vi "HFRR ADV v041.vi"() -> ()   [LabVIEW 2025] (continued)
                  frame False {
                  }
                  frame True {
                    w3298 = ";" ("Substring")
                    # "Pid out/\nFreq response value"
                    n2711 = local write "act save time"(w3344) -> ()
                    n2712 = local read "FILE"() -> (w3292:string)
                    n2713 = call "file check.vi"("file name in"=w3292) -> ("error out"=w3295:errorcluster, "file name out"=w3290:string)  [unwired: 9 in]
                    n2714 = local read "LVDT STROKE"() -> (w3287:dbl)
                    n2715 = local read "Add up Stroke"() -> (w3285:dbl)
                    n2716 = call "FILE PATH CREATION.vi"("error in"=w3295, "FILE NAME :"=w3290) -> ("FILE OUT"=w3293:path)  [unwired: 8 in, 1 out]
                    n2717 = local read "STROKE Initialize"() -> (w3280:bool)
                    n2718 = Concatenate Strings(w3290, ".dgf" ("Substring")) -> (w3294:string)
                    n2719 = Subtract(x=w3287, y=w3285) -> (x-y=w3286:dbl)
                    n2720 = Absolute Value(x=w3286) -> (abs(x)=w3283:dbl)
                    n2721 = local read "FF 2"() -> (→"Frictional Force ( N )" →"Frictional Force ( N )":dbl)
                    n2722 = Build Path(base path=w3293, name or relative path=w3294) -> (appended path=w3289:path)
                    n2723 = flat-sequence {
                      tunnel: w3283 -> [w3349]
                      tunnel: [w3348] -> w3281
                      tunnel: w3280 -> [w3346]
                      tunnel: [w3351] -> w3282
                      tunnel: w3281 -> [w3351]
                      frame #0 {
                        n2724 = call <vilib>:"Mean PtByPt.vi"("x"=w3349, "sample length"="STROKE FILTER", "initialize"=w3346) -> ("mean"=w3348:dbl)  [unwired: 1 in, 1 out]
                      }
                      frame #1 {
                        "STROKE Initialize" <- FALSE ("STROKE Initialize")
                      }
                    }
                    n2725 = local read "COF 2"() -> (w3303:dbl)
                    "Coefficient of Friction" <- w3303
                    "COF 4" <- w3303
                    "Coefficient of Friction" <- w3303
                    n2726 = local read "TEMP"() -> (w3306:dbl)
                    "Temperature ( Deg C )" <- w3306
                    n2727 = local read "Humidity ( %RH )"() -> (w3305:dbl)
                    n2728 = local read "Frequency ( Hz )"() -> (w3312:dbl)
                    n2729 = local read "LVDT STROKE DISPLAY"() -> (w3284:dbl)
                    n2730 = local read "Elapsed time"() -> (w3337:dbl)
                    n2731 = local read "AIR TEMP"() -> (w3310:dbl)
                    n2732 = local read "PID-out"() -> (w3315:dbl)
                    n2733 = local write "Temperature ( Deg C )"(w3306) -> ()
                    n2734 = Number To Fractional String(number=w3284, width (-)=i16 9 ("precision (6)"), precision (6)=i16 6) -> (F-format string=w3330:string)  [unwired: 1 in]
                    n2735 = Number To Fractional String(number=w3310, width (-)=i16 9 ("precision (6)"), precision (6)=i16 3) -> (F-format string=w3329:string)  [unwired: 1 in]
                    n2736 = Number To Fractional String(number=w3306, width (-)=i16 9 ("precision (6)"), precision (6)=i16 3) -> (F-format string=w3326:string)  [unwired: 1 in]
                    n2737 = Number To Fractional String(number=w3305, width (-)=i16 9 ("precision (6)"), precision (6)=i16 3) -> (F-format string=w3323:string)  [unwired: 1 in]
                    n2738 = Number To Fractional String(number=0.0, width (-)=i16 9 ("precision (6)"), precision (6)=i16 3) -> (F-format string=w3320:string)  [unwired: 1 in]
                    n2739 = Number To Fractional String(number=w3315, width (-)=i16 9 ("precision (6)"), precision (6)=i16 3) -> (F-format string=w3316:string)  [unwired: 1 in]
                    n2740 = Number To Fractional String(number=w3312, width (-)=i16 9 ("precision (6)"), precision (6)=i16 3) -> (F-format string=w3311:string)  [unwired: 1 in]
                    n2741 = Number To Fractional String(number=w3303, width (-)=i16 9 ("precision (6)"), precision (6)=i16 6) -> (F-format string=w3338:string)  [unwired: 1 in]
                    n2742 = Number To Fractional String(number=w3337, width (-)=i16 14 ("precision (6)"), precision (6)=i16 3) -> (F-format string=w3339:string)  [unwired: 1 in]
                    n2743 = Bundle("y"=1.02, "LVDT STROKE DISPLAY"=w3284, "y"=0.98) -> (w3304:T31)  [unwired: 1 in]
                    n2744 = Number To Fractional String(number="Ambient Humidity :", width (-)=i16 9 ("precision (6)"), precision (6)=i16 6) -> (F-format string=w3296:string)  [unwired: 1 in]
                    n2745 = local read "RUN"() -> (w3302:bool)
                    n2746 = case shown="True" w3302 {
                      tunnel: w3304 -> [_ w3355]
                      tunnel: w3284 -> [_ w3354]
                      tunnel: w3284 -> [_ w3352]
                      tunnel: w3284 -> [_ w3353]
                      frame False {
                      }
                      frame True {
                        "Stroke ( mm )" <- w3355
                        "Stroke ( mm )" <- w3355
                        "Stroke 4" <- w3354
                        "Stroke 3" <- w3352
                        "Stroke 2" <- w3353
                        "measured_stroke" <- w3352
                      }
                    }
                    n2747 = Concatenate Strings(w3339, w3298, w3338, w3298, w3330, w3298, w3329, w3298, w3326, w3298, w3323, w3298, w3320, w3298, w3316, w3298, w3311, w3298, w3296, "\r") -> (w3336:string)
                    n2748 = call <vilib>:"Write Characters To File.vi"("append to file? (new file:F)"=TRUE, "character string"=w3336, "file path (dialog if empty)"=w3289) -> ()  [unwired: 2 in, 1 out]
                    "refresh flag" <- TRUE ("refresh flag")
                    "LVDT STROKE Actual" <- w3282
                  }
                }
                n2749 = case shown="True" w3204 {
                  tunnel: w3214 -> [_ w3240]
                  tunnel: w3219 -> [_ w3250]
                  tunnel: [0.0 w3246] -> _
                  tunnel: w3213 -> [_ w3245]
                  tunnel: [0.0 w3244] -> _
                  tunnel: w3203 -> [_ w3244]
                  tunnel: w3217 -> [w3233 _]
                  frame False {
                    n2750 = local write "acq timer"(w3233) -> ()
                    n2751 = local write "Test Duration Status"(0.0 ("Test Duration Status")) -> ()
                  }
                  frame True {
                    n2752 = local read "Set Hz"() -> (w3247:dbl)
                    n2753 = local write "Elapsed time"(w3240) -> ()
                    n2754 = local read "test time"() -> (w3239:dbl)
                    n2755 = Multiply(x=w3250, y=w3247) -> (x*y=w3249:dbl)
                    n2756 = case shown="False" w3245 {
                      tunnel: w3249 -> [w3251 _]
                      tunnel: [w3251 1.0] -> w3246
                      frame False {
                        n2757 = local write "Cycles elapsed"(w3251) -> ()
                      }
                      frame True {
                      }
                    }
                    n2758 = Greater?(x=w3240, y=w3239) -> (0:w3248:bool)
                    n2759 = Subtract(x=w3239, y=w3240) -> (x-y=w3238:dbl)
                    n2760 = Multiply(x=w3238, y=60.0) -> (x*y=w3237:dbl)
                    n2761 = local write "Time Remaining"(w3237) -> ()
                    n2762 = local write "Remaining Time"(w3237) -> ()
                    n2763 = case shown="True" w3248 {
                      frame False {
                      }
                      frame True {
                        n2764 = stacked-sequence {
                          frame #0 {
                            w3256 = T19."Enabled" ("Disabled")
                            w3255 = FALSE ("TEST FILE NAM,E SAVED")
                            w3257 = "" ("FILE")
                            w3258 = TRUE ("Visible")
                            n2765 = local write "Humidity"(FALSE ("Humidity")) -> ()
                            n2766 = local write "RUN"(FALSE ("OK Button 2")) -> ()
                            n2767 = local write "Heater Button"(FALSE ("Heater Button")) -> ()
                            n2768 = local write "Auto Start Test"(FALSE ("Auto Start Test")) -> ()
                            n2769 = local write "TestCompFlg"(TRUE ("StpFlg")) -> ()
                            n2770 = local read "Humidity ( %RH )"() -> (→"Rh After":dbl)
                            n2771 = property on="STOP 2" class="Bool (strict)"("Disabled"=u8 0) -> ()  [unwired: 2 in, 2 out]
                            n2772 = local read "EVENT LOG"() -> (w3263:string)
                            n2773 = call "Event Log.vi"("Content"="Test Completed", "EVENT LOG"=w3263) -> ("EVENT LOG"=w3262:string)  [unwired: 8 in, 1 out]
                            n2774 = property on="RUN" class="Bool (strict)"("Visible"=w3258) -> ()  [unwired: 2 in, 2 out]
                            n2775 = property on="Auto Start Test" class="Bool (strict)"("Visible"=w3258) -> ()  [unwired: 2 in, 2 out]
                            n2776 = local write "Batch Ref Num :"(w3257) -> ()
                            n2777 = local write "FILE"(w3257) -> ()
                            n2778 = local write "EVENT LOG"(w3262) -> ()
                            n2779 = local write "TEST FILE NAM,E SAVED"(w3255) -> ()
                            n2780 = local write "Fuel Discription :"(w3257) -> ()
                            n2781 = local write "START TEMP"(w3255) -> ()
                            n2782 = local write "Remarks :"(w3257) -> ()
                            n2783 = local write "Main Dashboard Buttons"(T1."Imaging" ("Main Dashboard Buttons")) -> ()
                            n2784 = local write "Main Tab"(T2."Adv Scar" ("Main Tab")) -> ()
                            n2785 = property on="FRICVALZ 2" class="Bool (strict)"("DisabledEnum"=w3256) -> ()  [unwired: 2 in, 2 out]
                            n2786 = property on="FRICVALZ 3" class="Bool (strict)"("DisabledEnum"=w3256) -> ()  [unwired: 2 in, 2 out]
                            n2787 = property on="FRICVALZ 4" class="Bool (strict)"("DisabledEnum"=w3256) -> ()  [unwired: 2 in, 2 out]
                          }
                          frame #1 {
                            n2788 = Wait (ms)(milliseconds to wait=u32 1500) -> ()  [unwired: 1 out]
                          }
                          frame #2 {
                            n2789 = local write "Due Write"("VC;0") -> ()
                          }
                          frame #3 {
                            n2790 = Wait (ms)(milliseconds to wait=u32 1500) -> ()  [unwired: 1 out]
                          }
                          frame #4 {
                            n2791 = local write "Due Write"("VC;0") -> ()
                          }
                          frame #5 {
                            n2792 = Wait (ms)(milliseconds to wait=u32 1500) -> ()  [unwired: 1 out]
                          }
                          frame #6 {
                            n2793 = local write "Due Write"("ST;0") -> ()
                          }
                          frame #7 {
                            n2794 = local write "measured_stroke"(0.0 ("measured_stroke")) -> ()
                            n2795 = Wait (ms)(milliseconds to wait=u32 1500) -> ()  [unwired: 1 out]
                          }
                          frame #8 {
                            n2796 = local write "Due Write"("HE;0") -> ()
                            n2797 = local write "Humidity 2"(TRUE ("Humidity")) -> ()
                          }
                        }
                      }
                    }
                    n2798 = Divide(x=w3240, y=w3239) -> (x/y=w3243:dbl)
                    n2799 = Multiply(x=w3243, y=100.0) -> (x*y=w3241:dbl)
                    n2800 = local write "Test Duration Status"(w3241) -> ()
                  }
                }
              }
              frame #2 {
                n2801 = case shown="True" "Heater Button" {
                  tunnel: [0.0 ("output") w3378] -> w3356
                  frame False {
                    w3359 = TRUE ("tmpchk")
                    n2802 = local read "TEMP"() -> (w3360:dbl)
                    n2803 = local write "Temp ini"(w3360) -> ()
                    n2804 = local write "Reset 4"(w3359) -> ()
                    n2805 = local write "tmpchk"(w3359) -> ()
                    n2806 = local write "reinit"(TRUE ("reinit")) -> ()
                    n2807 = local write "manual temp log"(TRUE ("manual temp log")) -> ()
                  }
                  frame True {
                    # "Logic to turn off\nthe heater when \ntemp is not rising.\nTime - 60 sec\nDelta t- 5°c"
                    n2808 = local read "Temp ini"() -> (w3367:dbl)
                    n2809 = local read "Auto Start Test"() -> (w3363:bool)
                    n2810 = Less?(x=w3367, y=53.0) -> (x < y?=w3365:bool)
                    n2811 = case shown="False" w3363 {
                      frame False {
                        n2812 = local read "Set Temp"() -> (w3387:dbl)
                        n2813 = local read "TEMP"() -> (w3386:dbl)
                        n2814 = Subtract(x=w3387, y=w3386) -> (x-y=w3385:dbl)
                        n2815 = Absolute Value(x=w3385) -> (abs(x)=w3384:dbl)
                        n2816 = Less?(x=w3384, y=0.5) -> (x < y?=w3382:bool)
                        n2817 = case shown="True" w3382 {
                          tunnel: "manual temp log" -> [_ w3388]
                          frame False {
                          }
                          frame True {
                            n2818 = case shown="True" w3388 {
                              selector: w3388 -> [_ w3389]
                              frame False {
                              }
                              frame True {
                                # "#Event log"
                                n2819 = Not(x=w3389) -> (.not. x?=w3390:bool)
                                n2820 = local write "manual temp log"(w3390) -> ()
                                n2821 = local read "EVENT LOG"() -> (w3393:string)
                                n2822 = call "Event Log.vi"("Content"="Target Temperature reached", "EVENT LOG"=w3393) -> ("EVENT LOG"=w3392:string)  [unwired: 8 in, 1 out]
                                n2823 = local write "EVENT LOG"(w3392) -> ()
                              }
                            }
                          }
                        }
                      }
                      frame True {
                        n2824 = local write "manual temp log"(TRUE ("manual temp log")) -> ()
                      }
                    }
                    n2825 = And(x="tmpchk", y=w3365) -> (x .and. y?=w3368:bool)
                    n2826 = case shown="True" w3368 {
                      frame False {
                      }
                      frame True {
                        n2827 = call "Elapsed Time8"("Time Target (s)"=300.0, "Reset"="Reset 4") -> ("Time has Elapsed"=w3395:bool)  [unwired: 10 in, 7 out]
                        n2828 = flat-sequence {
                          tunnel: w3395 -> [_]
                          frame #0 {
                            n2829 = local write "Reset 4"(FALSE ("Reset 4")) -> ()
                          }
                        }
                        n2830 = case shown="True" w3395 {
                          frame False {
                          }
                          frame True {
                            n2831 = local read "Temp ini"() -> (w3402:dbl)
                            n2832 = Add(x=w3402, y=5.0) -> (x+y=w3400:dbl)
                            n2833 = local read "TEMP"() -> (w3403:dbl)
                            n2834 = Greater?(x=w3403, y=w3400) -> (0:w3401:bool)
                            n2835 = case shown="False" w3401 {
                              frame False {
                                n2836 = local write "Heater Button"(FALSE ("Heater Button")) -> ()
                              }
                              frame True {
                                n2837 = local write "tmpchk"(FALSE ("tmpchk")) -> ()
                              }
                            }
                          }
                        }
                      }
                    }
                    n2838 = local read "Set Temp"() -> (w3376:dbl)
                    n2839 = local read "TEMP"() -> (w3370:dbl)
                    n2840 = call-poly <vilib>:"PID.vi"("reinitialize? (F)"="reinit", "dt (s)"=-1.0, "process variable"=w3370, "setpoint"=w3376) -> ("output"=w3373:dbl)  [unwired: 6 in, 1 out]
                    n2841 = Subtract(x=w3376, y=w3370) -> (x-y=w3377:dbl)
                    n2842 = Add(x=w3376, y=0.5) -> (x+y=w3374:dbl)
                    n2843 = Greater Or Equal?(x=w3370, y=w3374) -> ()  [unwired: 1 out]
                    n2844 = Select(t=0.0, s=FALSE, f=w3373) -> (s? t:f=w3372:dbl)
                    "PID output" <- w3372
                    n2845 = flat-sequence {
                      tunnel: w3372 -> [w3406]
                      tunnel: [w3406] -> w3378
                      frame #0 {
                        n2846 = local write "reinit"(FALSE ("reinit")) -> ()
                      }
                    }
                    n2847 = Bundle(w3377, "output"=w3372, "TEMP"=w3370) -> ()  [unwired: 1 in, 1 out]
                  }
                }
                "PID-out" <- w3356
              }
              frame #3 {
                n2848 = local read "TEMP"() -> (w3408:dbl)
                n2849 = Greater Or Equal?(x=w3408, y="Set Temp 2") -> (x >= y?=w3413:bool)
                n2850 = case shown="True" w3413 {
                  tunnel: [FALSE TRUE] -> w3411
                  frame False {
                  }
                  frame True {
                  }
                }
                "Status 13" <- w3411
                n2851 = And(x=w3411, y="trip1 8") -> (x .and. y?=w3410:bool)
                n2852 = case shown="True" w3410 {
                  frame False {
                    n2853 = local write "Heater Trip Temp"(TRUE ("Heater Trip Temp")) -> ()
                  }
                  frame True {
                    w3416 = FALSE ("OK Button 2")
                    n2854 = case shown="True" "Heater Trip Temp" {
                      selector: "Heater Trip Temp" -> [_ w3418]
                      frame False {
                      }
                      frame True {
                        n2855 = Not(x=w3418) -> (.not. x?=w3417:bool)
                        n2856 = local read "EVENT LOG"() -> (w3421:string)
                        n2857 = local write "Heater Trip Temp"(w3417) -> ()
                        n2858 = call "Event Log.vi"("Content"="Heater Trip", "EVENT LOG"=w3421) -> ("EVENT LOG"=w3420:string)  [unwired: 8 in, 1 out]
                        n2859 = local write "EVENT LOG"(w3420) -> ()
                      }
                    }
                    n2860 = local write "RUN"(w3416) -> ()
                    n2861 = property on="Auto Start Test" class="Bool (strict)"("Value"=w3416) -> ()  [unwired: 2 in, 2 out]
                    n2862 = local write "Heater Button"(w3416) -> ()
                  }
                }
              }
            }
            n2863 = case shown="False" w3127 {
              frame False {
                n2864 = disable-structure shown="Disabled" {
                  frame Disabled {
                    n2865 = stacked-sequence {
                      frame #0 {
                        n2866 = local write "RUN"(FALSE ("OK Button 2")) -> ()
                      }
                      frame #1 {
                      }
                    }
                  }
                  frame Enabled {
                  }
                }
              }
              frame True {
              }
            }
          }
        }
        n2867 = local read "Reset Graph"() -> (w3024:bool)
        n2868 = case shown="True" w3024 {
          selector: w3024 -> [_ w3041]
          frame False {
          }
          frame True {
            w3055 = 0.0 ("X Scale.Range:Maximum")
            n2869 = Not(x=w3041) -> (.not. x?=w3040:bool)
            n2870 = local write "Reset Graph"(w3040) -> ()
            n2871 = property on="Electrical Contact Resistance ( % )" class="WFChart (strict)"("XScale.Maximum"=600.0 ("X Scale.Range:Maximum"), "XScale.Minimum"=0.0 ("X Scale.Range:Minimum"), "YScale.Maximum"=100.0 ("Y Scale.Range:Maximum"), "YScale.Minimum"=0.0 ("Y Scale.Range:Minimum")) -> ()  [unwired: 2 in, 2 out]
            n2872 = property on="Frictional Force ( N )" class="WFChart (strict)"("XScale.Maximum"=600.0 ("X Scale.Range:Maximum"), "XScale.Minimum"=0.0 ("X Scale.Range:Minimum"), "YScale.Maximum"=100.0 ("Y Scale.Range:Maximum"), "YScale.Minimum"=0.0 ("Y Scale.Range:Minimum")) -> ()  [unwired: 2 in, 2 out]
            n2873 = property on="Temperature ( Deg C )" class="WFChart (strict)"("XScale.Maximum"=600.0 ("X Scale.Range:Maximum"), "XScale.Minimum"=0.0 ("X Scale.Range:Minimum"), "YScale.Maximum"=100.0 ("Y Scale.Range:Maximum"), "YScale.Minimum"=0.0 ("Y Scale.Range:Minimum")) -> ()  [unwired: 2 in, 2 out]
            n2874 = property on="Stroke ( mm )" class="WFChart (strict)"("XScale.Maximum"=600.0 ("X Scale.Range:Maximum"), "XScale.Minimum"=0.0 ("X Scale.Range:Minimum"), "YScale.Maximum"=100.0 ("Y Scale.Range:Maximum"), "YScale.Minimum"=0.0 ("Y Scale.Range:Minimum")) -> ()  [unwired: 2 in, 2 out]
            n2875 = property on="Coefficient of Friction" class="WFChart (strict)"("XScale.Maximum"=600.0 ("X Scale.Range:Maximum"), "XScale.Minimum"=0.0 ("X Scale.Range:Minimum"), "YScale.Maximum"=100.0 ("Y Scale.Range:Maximum"), "YScale.Minimum"=0.0 ("Y Scale.Range:Minimum")) -> ()  [unwired: 2 in, 2 out]
            n2876 = property on="Electrical Contact Resistance ( % )" class="WFChart (strict)"("XScale.Minimum"=0.0 ("X Scale.Range:Minimum"), "XScale.Maximum"=600.0 ("X Scale.Range:Maximum"), "YScale.Minimum"=0.0 ("Y Scale.Range:Minimum"), "YScale.Maximum"=100.0 ("Y Scale.Range:Maximum")) -> ()  [unwired: 2 in, 2 out]
            n2877 = property on="Temperature ( Deg C )" class="WFChart (strict)"("XScale.Minimum"=0.0 ("X Scale.Range:Minimum"), "XScale.Maximum"=600.0 ("X Scale.Range:Maximum"), "YScale.Minimum"=0.0 ("Y Scale.Range:Minimum"), "YScale.Maximum"=100.0 ("Y Scale.Range:Maximum")) -> ()  [unwired: 2 in, 2 out]
            n2878 = property on="Coefficient of Friction" class="WFChart (strict)"("XScale.Minimum"=0.0 ("X Scale.Range:Minimum"), "XScale.Maximum"=600.0 ("X Scale.Range:Maximum"), "YScale.Maximum"=1.0 ("X Scale.Range:Minimum"), "YScale.Minimum"=0.0 ("X Scale.Range:Minimum")) -> ()  [unwired: 2 in, 2 out]
            n2879 = property on="Frictional Force ( N )" class="WFChart (strict)"("XScale.Maximum"=600.0 ("X Scale.Range:Maximum"), "XScale.Minimum"=w3055, "YScale.Maximum"=10.0 ("Y Scale.Range:Maximum"), "YScale.Minimum"=w3055) -> ()  [unwired: 2 in, 2 out]
            n2880 = property on="Stroke ( mm )" class="WFChart (strict)"("XScale.Maximum"=600.0 ("X Scale.Range:Maximum"), "XScale.Minimum"=0.0 ("X Scale.Range:Minimum"), "YScale.Maximum"=100.0 ("Y Scale.Range:Maximum"), "YScale.Minimum"=0.0 ("Y Scale.Range:Minimum")) -> ()  [unwired: 2 in, 2 out]
          }
        }
      }
      frame "Compare Files" {
        # "Elapsed time\ncof\nstroke\nAir temp\nTemp\nHumidity"
        n2881 = case shown="True" "RSTV1 2" {
          frame False {
          }
          frame True {
            n2882 = property on="Humidity ( %RH )" class="XYGraph (strict)"("Y Scale.Display Format:Precision"=u8 0 ("Y Scale.Format & Precision:Precision")) -> ()  [unwired: 2 in, 2 out]
            n2883 = property on="Humidity ( %RH )" class="XYGraph (strict)"("X Scale.Range:Minimum"=0.0, "X Scale.Range:Maximum"=75.0, "Y Scale.Range:Minimum"=48.0, "Y Scale.Range:Maximum"=58.0) -> ()  [unwired: 2 in, 2 out]
          }
        }
        n2884 = case shown="True" "RST CP 2" {
          frame False {
          }
          frame True {
            n2885 = property on="XY Graph 13" class="XYGraph (strict)"("Y Scale.Display Format:Precision"=u8 0 ("Y Scale.Format & Precision:Precision")) -> ()  [unwired: 2 in, 2 out]
            n2886 = property on="XY Graph 13" class="XYGraph (strict)"("X Scale.Range:Minimum"=0.0, "X Scale.Range:Maximum"=75.0, "Y Scale.Range:Minimum"=0.0, "Y Scale.Range:Maximum"=100.0) -> ()  [unwired: 2 in, 2 out]
          }
        }
        n2887 = case shown="True" "RST CP" {
          frame False {
          }
          frame True {
            n2888 = property on="Sample Temperature ( °C )" class="XYGraph (strict)"("Y Scale.Display Format:Precision"=u8 2 ("Y Scale.Format & Precision:Precision")) -> ()  [unwired: 2 in, 2 out]
            n2889 = property on="Sample Temperature ( °C )" class="XYGraph (strict)"("X Scale.Range:Minimum"=0.0, "X Scale.Range:Maximum"=75.0, "Y Scale.Range:Minimum"=58.0, "Y Scale.Range:Maximum"=62.0) -> ()  [unwired: 2 in, 2 out]
          }
        }
        n2890 = case shown="True" "RSTV1 3" {
          frame False {
          }
          frame True {
            n2891 = property on="Air Temperature  ( °C )" class="XYGraph (strict)"("Y Scale.Display Format:Precision"=u8 2 ("Y Scale.Format & Precision:Precision")) -> ()  [unwired: 2 in, 2 out]
            n2892 = property on="Air Temperature  ( °C )" class="XYGraph (strict)"("X Scale.Range:Minimum"=0.0 ("Y Scale.Range:Minimum"), "X Scale.Range:Maximum"=75.0 ("Y Scale.Range:Maximum"), "Y Scale.Range:Minimum"=20.0 ("X Scale.Range:Minimum"), "Y Scale.Range:Maximum"=26.0 ("X Scale.Range:Maximum")) -> ()  [unwired: 2 in, 2 out]
          }
        }
        n2893 = case shown="True" "RSTV1 4" {
          frame False {
          }
          frame True {
            n2894 = property on="Stroke ( mm )" class="XYGraph (strict)"("Y Scale.Display Format:Precision"=u8 2 ("Y Scale.Format & Precision:Precision")) -> ()  [unwired: 2 in, 2 out]
            n2895 = property on="Stroke ( mm )" class="XYGraph (strict)"("X Scale.Range:Minimum"=0.0 ("Y Scale.Range:Maximum"), "X Scale.Range:Maximum"=75.0 ("X Scale.Range:Minimum"), "Y Scale.Range:Minimum"=0.98, "Y Scale.Range:Maximum"=1.02) -> ()  [unwired: 2 in, 2 out]
          }
        }
        n2896 = case shown="True" "rstv2" {
          frame False {
          }
          frame True {
            n2897 = property on="Coefficient Of Friction" class="XYGraph (strict)"("Y Scale.Display Format:Precision"=u8 3 ("Y Scale.Format & Precision:Precision")) -> ()  [unwired: 2 in, 2 out]
            n2898 = property on="Coefficient Of Friction" class="XYGraph (strict)"("X Scale.Range:Minimum"=0.0 ("Y Scale.Range:Maximum"), "X Scale.Range:Maximum"=75.0, "Y Scale.Range:Minimum"=0.0, "Y Scale.Range:Maximum"=1.0 ("X Scale.Range:Minimum")) -> ()  [unwired: 2 in, 2 out]
          }
        }
        n2899 = case shown="True" "RST CP 3" {
          frame False {
          }
          frame True {
            n2900 = property on="Air Temp ( °C ) vs Humidity ( % RH )" class="XYGraph (strict)"("X Scale.Range:Minimum"=18.0, "X Scale.Range:Maximum"=28.0 ("X Scale.Range:Minimum"), "Y Scale.Range:Minimum"=30.0 ("X Scale.Range:Minimum"), "Y Scale.Range:Maximum"=70.0 ("X Scale.Range:Minimum")) -> ()  [unwired: 2 in, 2 out]
          }
        }
        n2901 = case shown="True" "OPEN 1" {
          frame False {
          }
          frame True {
            (unwired) 0  # existing file
            w3697 = "Choose a datalog file to open"  # prompt
            n2902 = local write "OPEN 1"(FALSE ("OPEN 1")) -> ()
            n2903 = String To Path(string="C:\\LAB-IQ\\Data\\") -> (path=w3682:path)
            n2904 = File Dialog(6:"*.dgf" ("pattern"), 7:w3697, 11:w3682) -> (0:w3680:errorcluster, 3:w3688:path)  [unwired: 4 in, 2 out]
            n2905 = Unbundle(w3680) -> ()  [unwired: 3 out]
            n2906 = Strip Path(path=w3688) -> (name=w3687:string)  [unwired: 1 out]
            n2907 = Path To String(path=w3688) -> (string=w3683:string)
            "string1" <- w3683
            n2908 = Match Pattern(string=w3687, regular expression=".dgf") -> (before substring=→"String Control":string)  [unwired: 1 in, 3 out]
            n2909 = Match Pattern(string=w3683, regular expression=".dgf" ("substring (\"\")")) -> (before substring=w3693:string)  [unwired: 1 in, 3 out]
            n2910 = Concatenate Strings(w3693, ".duf" ("Substring")) -> (w3689:string)
            n2911 = String To Path(string=w3689) -> (path=w3694:path)
            n2912 = call <vilib>:"Read Characters From File.vi"("file path (dialog if empty)"=w3694, "start of read offset (chars.:0)"=60 ("start of read offset (chars.: 0)")) -> ("character string"=→"String Control 2":string)  [unwired: 4 in, 3 out]
          }
        }
        n2913 = case shown="True" "OPEN 2" {
          frame False {
          }
          frame True {
            (unwired) 0  # existing file
            w3715 = "Choose a datalog file to open"  # prompt
            n2914 = local write "OPEN 2"(FALSE ("OPEN 1")) -> ()
            n2915 = String To Path(string="C:\\LAB-IQ\\Data\\") -> (path=w3700:path)
            n2916 = File Dialog(6:"*.dgf" ("pattern"), 7:w3715, 11:w3700) -> (0:w3698:errorcluster, 3:w3706:path)  [unwired: 4 in, 2 out]
            n2917 = Unbundle(w3698) -> ()  [unwired: 3 out]
            n2918 = Strip Path(path=w3706) -> (name=w3704:string)  [unwired: 1 out]
            n2919 = Path To String(path=w3706) -> (string=w3701:string)
            "string1 2" <- w3701
            n2920 = Match Pattern(string=w3704, regular expression=".dgf") -> (before substring=→"String Control 3":string)  [unwired: 1 in, 3 out]
            n2921 = Match Pattern(string=w3701, regular expression=".dgf" ("substring (\"\")")) -> (before substring=w3712:string)  [unwired: 1 in, 3 out]
            n2922 = Concatenate Strings(w3712, ".duf" ("Substring")) -> (w3709:string)
            n2923 = String To Path(string=w3709) -> (path=w3707:path)
            n2924 = call <vilib>:"Read Characters From File.vi"("file path (dialog if empty)"=w3707, "start of read offset (chars.:0)"=60 ("start of read offset (chars.: 0)")) -> ("character string"=→"String Control 4":string)  [unwired: 4 in, 3 out]
          }
        }
        n2925 = case shown="True" "OPEN 3" {
          frame False {
          }
          frame True {
            (unwired) 0  # existing file
            w3733 = "Choose a datalog file to open"  # prompt
            n2926 = local write "OPEN 3"(FALSE ("OPEN 1")) -> ()
            n2927 = String To Path(string="C:\\LAB-IQ\\Data\\") -> (path=w3718:path)
            n2928 = File Dialog(6:"*.dgf" ("pattern"), 7:w3733, 11:w3718) -> (0:w3716:errorcluster, 3:w3724:path)  [unwired: 4 in, 2 out]
            n2929 = Unbundle(w3716) -> ()  [unwired: 3 out]
            n2930 = Strip Path(path=w3724) -> (name=w3722:string)  [unwired: 1 out]
            n2931 = Path To String(path=w3724) -> (string=w3719:string)
            "string1 3" <- w3719
            n2932 = Match Pattern(string=w3722, regular expression=".dgf") -> (before substring=→"String Control 5":string)  [unwired: 1 in, 3 out]
            n2933 = Match Pattern(string=w3719, regular expression=".dgf" ("substring (\"\")")) -> (before substring=w3729:string)  [unwired: 1 in, 3 out]
            n2934 = Concatenate Strings(w3729, ".duf" ("Substring")) -> (w3726:string)
            n2935 = String To Path(string=w3726) -> (path=w3730:path)
            n2936 = call <vilib>:"Read Characters From File.vi"("file path (dialog if empty)"=w3730, "start of read offset (chars.:0)"=60 ("start of read offset (chars.: 0)")) -> ("character string"=→"String Control 6":string)  [unwired: 4 in, 3 out]
          }
        }
        n2937 = case shown="True" "OPEN 4" {
          frame False {
          }
          frame True {
            (unwired) 0  # existing file
            w3751 = "Choose a datalog file to open"  # prompt
            n2938 = local write "OPEN 4"(FALSE ("OPEN 1")) -> ()
            n2939 = String To Path(string="C:\\LAB-IQ\\Data\\") -> (path=w3736:path)
            n2940 = File Dialog(6:"*.dgf" ("pattern"), 7:w3751, 11:w3736) -> (0:w3734:errorcluster, 3:w3742:path)  [unwired: 4 in, 2 out]
            n2941 = Unbundle(w3734) -> ()  [unwired: 3 out]
            n2942 = Strip Path(path=w3742) -> (name=w3740:string)  [unwired: 1 out]
            n2943 = Path To String(path=w3742) -> (string=w3737:string)
            "string1 4" <- w3737
            n2944 = Match Pattern(string=w3740, regular expression=".dgf") -> (before substring=→"String Control 7":string)  [unwired: 1 in, 3 out]
            n2945 = Match Pattern(string=w3737, regular expression=".dgf" ("substring (\"\")")) -> (before substring=w3747:string)  [unwired: 1 in, 3 out]
            n2946 = Concatenate Strings(w3747, ".duf" ("Substring")) -> (w3744:string)
            n2947 = String To Path(string=w3744) -> (path=w3748:path)
            n2948 = call <vilib>:"Read Characters From File.vi"("file path (dialog if empty)"=w3748, "start of read offset (chars.:0)"=60 ("start of read offset (chars.: 0)")) -> ("character string"=→"String Control 8":string)  [unwired: 4 in, 3 out]
          }
        }
      }
      frame "About" {
        # "Elapsed time\ncof\nstroke\nmean pos\nTemp\nHumidity"
        n2949 = disable-structure shown="Disabled" {
          frame Disabled {
            n2950 = case shown="True" "Export" {
              frame False {
              }
              frame True {
                w3773 = "                                      " ("string")
                w3775 = "\r"
                (unwired) i16 6 ("width (-)")
                w3852 = "\r"
                w3784 = "\r"
                n2951 = local write "Export"(FALSE ("Export")) -> ()
                n2952 = local read "String 29"() -> (w3821:string)
                n2953 = local read "String 34"() -> (w3809:string)
                n2954 = local read "String 35"() -> (w3804:string)
                n2955 = local read "String 37"() -> (w3800:string)
                n2956 = local read "String 36"() -> (w3797:string)
                n2957 = local read "String 38"() -> (w3794:string)
                n2958 = local read "String 39"() -> (w3791:string)
                n2959 = Match Pattern(string=w3821, regular expression=".dwm") -> (before substring=w3817:string)  [unwired: 1 in, 3 out]
                "before substring" <- w3817
                n2960 = local read "S 38"() -> (w3812:string)
                n2961 = local read "S 39"() -> (w3805:string)
                n2962 = local read "Temperature before test 2"() -> (w3841:dbl)
                n2963 = local read "Temperature after test 2"() -> (w3846:dbl)
                n2964 = local read "Humidity before test 2"() -> (w3827:dbl)
                n2965 = local read "Humidity after test 2"() -> (w3842:dbl)
                n2966 = local read "MWSD 2"() -> (w3838:dbl)
                n2967 = local read "WS1.4 2"() -> (w3854:dbl)
                n2968 = local read "HCF 2"() -> (w3850:dbl)
                n2969 = local read "AVP 2"() -> (w3839:dbl)
                n2970 = Concatenate Strings("1," ("string"), w3812) -> (w3811:string)
                n2971 = Concatenate Strings("2," ("string"), w3809) -> (w3808:string)
                n2972 = Concatenate Strings("3," ("string"), w3805) -> (w3807:string)
                n2973 = Concatenate Strings("4," ("string"), w3804) -> (w3803:string)
                n2974 = Concatenate Strings("5," ("string"), w3800) -> (w3801:string)
                n2975 = Concatenate Strings("6," ("string"), w3797) -> (w3798:string)
                n2976 = Concatenate Strings("7," ("string"), w3794) -> (w3795:string)
                n2977 = Concatenate Strings("8," ("string"), w3791) -> (w3792:string)
                n2978 = local read "Sample ID"() -> (w3859:string)
                n2979 = case shown="\"xlx\"" "Select File Type" {
                  tunnel: w3817 -> [w3862 w3864 w3866]
                  tunnel: [w3860 w3865 w3867] -> w3816
                  frame "xlx" {
                    n2980 = Concatenate Strings(w3862, ".xls" ("string")) -> (w3860:string)
                  }
                  frame "csv" {
                    n2981 = Concatenate Strings(w3864, ".csv" ("string")) -> (w3865:string)
                  }
                  frame "txt" {
                    n2982 = Concatenate Strings(w3866, ".txt" ("string")) -> (w3867:string)
                  }
                }
                n2983 = local read "Test Date"() -> (w3858:string)
                n2984 = local read "String 45"() -> (w3772:string)
                n2985 = local read "String 31"() -> (w3857:string)
                n2986 = local read "String 32"() -> (w3856:string)
                n2987 = local read "TITTLE"() -> (w3780:string)
                n2988 = Number To Fractional String(number=w3827, width (-)=i16 6, precision (6)=i16 2) -> (F-format string=w3826:string)  [unwired: 1 in]
                n2989 = Number To Fractional String(number=w3841, width (-)=i16 6, precision (6)=i16 2) -> (F-format string=w3847:string)  [unwired: 1 in]
                n2990 = Number To Fractional String(number=w3842, width (-)=i16 6, precision (6)=i16 2) -> (F-format string=w3840:string)  [unwired: 1 in]
                n2991 = Number To Fractional String(number=w3846, width (-)=i16 6, precision (6)=i16 2) -> (F-format string=w3845:string)  [unwired: 1 in]
                n2992 = Number To Fractional String(number=w3838, width (-)=i16 6, precision (6)=i16 2) -> (F-format string=w3836:string)  [unwired: 1 in]
                n2993 = Number To Fractional String(number=w3839, width (-)=i16 6, precision (6)=i16 2) -> (F-format string=w3837:string)  [unwired: 1 in]
                n2994 = Number To Fractional String(number=w3850, width (-)=i16 6, precision (6)=i16 2) -> (F-format string=w3851:string)  [unwired: 1 in]
                n2995 = Number To Fractional String(number=w3854, precision (6)=i16 2) -> (F-format string=w3855:string)  [unwired: 2 in]
                n2996 = local read "s.NO"() -> (w3774:string)
                n2997 = Concatenate Strings("=" ("string"), w3780) -> (w3779:string)
                n2998 = Concatenate Strings("S.No," ("string"), "                                       Parameters" ("string")) -> (w3785:string)
                n2999 = Concatenate Strings(w3852, w3811, w3826, w3852, w3808, w3847, w3852, w3807, w3840, w3852, w3803, w3845, w3852, w3801, w3836, w3852, w3798, w3837, w3852, w3795, w3851, w3852, w3792, w3855) -> (w3814:string)
                n3000 = Concatenate Strings(w3784, "," ("string"), w3772, w3774, w3773, w3856, w3859, w3773, w3857, w3858, w3784) -> (w3782:string)
                n3001 = local read "Tested by"() -> (w3788:string)
                n3002 = local read "String 33"() -> (w3789:string)
                n3003 = Concatenate Strings("," ("string"), "                                                                             " ("string")) -> (w3777:string)
                n3004 = Concatenate Strings(w3779, w3775, w3782, w3775, w3785, w3814, w3775, w3777, w3789, w3788) -> (→"export":string)
                n3005 = String To Path(string=w3816) -> (path=w3823:path)
                n3006 = local read "export"() -> (w3818:string)
                n3007 = call <vilib>:"Write Characters To File.vi"("append to file? (new file:F)"=FALSE, "character string"=w3818, "file path (dialog if empty)"=w3823) -> ()  [unwired: 2 in, 1 out]
              }
            }
          }
          frame Enabled {
          }
        }
        n3008 = case shown="True" "OK Button 17" {
          frame False {
          }
          frame True {
            (unwired) 0  # existing file
            w4076 = "Choose a datalog file to open"  # prompt
            n3009 = local write "OK Button 17"(FALSE ("OK Button 17")) -> ()
            n3010 = local read "String"() -> (w4071:string)
            n3011 = String To Path(string=w4071) -> (path=w4072:path)
            n3012 = File Dialog(6:"*.duf" ("pattern"), 7:w4076, 11:w4072) -> (0:w4063:errorcluster, 3:w4082:path)  [unwired: 4 in, 2 out]
            n3013 = Unbundle(w4063) -> ()  [unwired: 3 out]
            n3014 = Open/Create/Replace File "Open File"(file path (use dialog)=w4082) -> (refnum out=w4074:refnum<file>)  [unwired: 5 in, 2 out]
            n3015 = Strip Path(path=w4082) -> (name=w4080:string)  [unwired: 1 out]
            n3016 = Path To String(path=w4082) -> (string=w4065:string)
            n3017 = while {
              tunnel: w4074 -> [w4086]
              i -> [w4083]
              stop <- w4084 continue-if-true
              (unwired) TRUE ("line mode (F)")
              n3018 = Read from Text File "Read File"(file (use dialog)=w4086) -> (text=w4085:string)  [unwired: 3 in, 3 out]
              n3019 = local write "Numeric 16"(w4083) -> ()
              n3020 = String Length(string=w4085) -> (length=w4088:i32)
              n3021 = Greater?(x=w4088, y=1) -> (0:w4084:bool)
            }
            n3022 = local write "String 29"(w4065) -> ()
            n3023 = Search and Replace String(input string=w4065, search string=".duf", replace string=".dgf" ("replace string (\"\")")) -> (result string=→"String Indicator 4":string)  [unwired: 5 in, 3 out]
            n3024 = Match Pattern(string=w4080, regular expression=".dwm") -> (before substring=w4064:string)  [unwired: 1 in, 3 out]
            "String Indicator" <- w4064
            n3025 = Match Pattern(string=w4065, regular expression=".dwm" ("substring (\"\")")) -> (before substring=w4066:string)  [unwired: 1 in, 3 out]
            "String Indicator 3" <- w4066
            n3026 = local write "TITTLE 2"(w4064) -> ()
            n3027 = String To Path(string=w4066) -> (path=w4073:path)
            "path" <- w4073
            n3028 = call <vilib>:"Read Characters From File.vi"("file path (dialog if empty)"=w4073, "start of read offset (chars.:0)"=60 ("start of read offset (chars.: 0)")) -> ("character string"=→"String Indicator 2":string)  [unwired: 4 in, 3 out]
          }
        }
        n3029 = call <vilib>:"Query Available Printers.vi"() -> ("system configured printers"=w3765:string[])  [unwired: 9 in, 2 out]
        "System Configured Printers 2" <- w3765
        n3030 = local read "OK Button 16"() -> (w3762:bool)
        n3031 = case shown="True" "OK Button 16" {
          frame False {
          }
          frame True {
            n3032 = stacked-sequence {
              frame #0 {
                n3033 = local read "Numeric 16"() -> (w4090:i32)
                n3034 = local write "Numeric 10"(w4090) -> ()
              }
              frame #1 {
                n3035 = local read "String 29"() -> (w4093:string)
                n3036 = String To Path(string=w4093) -> (path=w4092:path)
                n3037 = Open/Create/Replace File "Open File"(file path (use dialog)=w4092) -> (refnum out=w4094:refnum<file>)  [unwired: 5 in, 2 out]
                n3038 = for {
                  N: 16 -> [_]
                  tunnel: w4094 -> [w4101]
                  i -> [w4097]
                  (unwired) TRUE ("line mode (F)")
                  n3039 = Read from Text File "Read File"(file (use dialog)=w4101) -> (text=w4095:string)  [unwired: 3 in, 3 out]
                  n3040 = Match Pattern(string=w4095, regular expression="(") -> (after substring=w4100:string)  [unwired: 1 in, 3 out]
                  n3041 = Match Pattern(string=w4100, regular expression=")") -> (before substring=w4096:string)  [unwired: 1 in, 3 out]
                  n3042 = case shown="1" w4097 {
                    tunnel: w4096 -> [w4102 w4103 _ _ w4104 w4105 w4106 w4108 w4110 w4112 w4114 w4116 w4118 w4120 _]
                    tunnel: w4095 -> [_ _ _ _ _ _ _ _ _ _ _ _ _ _ _]
                    frame 0 {
                      "TITTLE" <- w4102
                    }
                    frame 1 {
                      "Sample ID" <- w4103
                    }
                    frame 2 {
                    }
                    frame 3 {
                    }
                    frame 4 {
                      "Test Date" <- w4104
                    }
                    frame 5 {
                      "Tested by" <- w4105
                    }
                    frame 6 {
                      n3043 = Fract/Exp String To Number(string=w4106) -> (number=→"Humidity before test 2":dbl)  [unwired: 3 in, 1 out]
                    }
                    frame 7 {
                      n3044 = Fract/Exp String To Number(string=w4108) -> (number=→"Temperature before test 2":dbl)  [unwired: 3 in, 1 out]
                    }
                    frame 8 {
                      n3045 = Fract/Exp String To Number(string=w4110) -> (number=→"Humidity after test 2":dbl)  [unwired: 3 in, 1 out]
                    }
                    frame 9 {
                      n3046 = Fract/Exp String To Number(string=w4112) -> (number=→"Temperature after test 2":dbl)  [unwired: 3 in, 1 out]
                    }
                    frame 10 {
                      n3047 = Fract/Exp String To Number(string=w4114) -> (number=→"MWSD 2":dbl)  [unwired: 3 in, 1 out]
                    }
                    frame 11 {
                      n3048 = Fract/Exp String To Number(string=w4116) -> (number=→"AVP 2":dbl)  [unwired: 3 in, 1 out]
                    }
                    frame 12 {
                      n3049 = Fract/Exp String To Number(string=w4118) -> (number=→"HCF 2":dbl)  [unwired: 3 in, 1 out]
                    }
                    frame 13 {
                      n3050 = Fract/Exp String To Number(string=w4120) -> (number=→"WS1.4 2":dbl)  [unwired: 3 in, 1 out]
                    }
                    frame 14, Default {
                    }
                  }
                }
              }
              frame #2 {
              }
            }
            n3051 = local write "OK Button 16"(FALSE ("OK Button 13")) -> ()
          }
        }
        n3052 = Index Array(array=w3765, index="Select Printer 3") -> (element=w3767:string)
        "Selected Printer" <- w3767
        n3053 = case shown="True" w3762 {
          frame False {
          }
          frame True {
            n3054 = flat-sequence {
              frame #0 {
              }
              frame #1 {
                n3055 = Wait (ms)(milliseconds to wait=u32 100) -> ()  [unwired: 1 out]
              }
              frame #2 {
                n3056 = local write "OK Button 16"(FALSE ("Print 3")) -> ()
              }
            }
          }
        }
        n3057 = case shown="True" "Print" {
          tunnel: w3767 -> [_ w4059]
          frame False {
          }
          frame True {
            (unwired) i16 6 ("width (-)")
            (unwired) "TESTED BY : "
            (unwired) "TESTED DATE :"
            (unwired) "SAMPLE ID : "
            (unwired) "SAMPLE DESIGN : "
            w4017 = "\r"
            w4034 = "\r"
            # "add image"
            n3058 = local read "Sample ID"() -> (w4007:string)
            n3059 = local read "Tested by"() -> (w4010:string)
            n3060 = local read "String 34"() -> (w3997:string)
            n3061 = local read "String 45"() -> (w3977:string)
            n3062 = local read "String 35"() -> (w3992:string)
            n3063 = local read "String 37"() -> (w3990:string)
            n3064 = local read "String 32"() -> (w4012:string)
            n3065 = local read "String 36"() -> (w3987:string)
            n3066 = local read "String 31"() -> (w4011:string)
            n3067 = local read "Test Date"() -> (w4008:string)
            n3068 = local read "String 33"() -> (w4013:string)
            n3069 = local read "String 38"() -> (w3983:string)
            n3070 = local read "String 39"() -> (w3980:string)
            n3071 = local write "Print"(FALSE ("Print FF")) -> ()
            n3072 = local read "S 39"() -> (w3995:string)
            n3073 = local read "S 38"() -> (w4002:string)
            n3074 = local read "Temperature before test 2"() -> (w4033:dbl)
            n3075 = local read "Temperature after test 2"() -> (w4023:dbl)
            n3076 = local read "Humidity before test 2"() -> (w4048:dbl)
            n3077 = local read "Humidity after test 2"() -> (w4032:dbl)
            n3078 = local read "MWSD 2"() -> (w4037:dbl)
            n3079 = local read "WS1.4 2"() -> (w4015:dbl)
            n3080 = Concatenate Strings("2)" ("string"), w3997) -> (w3998:string)
            n3081 = Concatenate Strings("3)" ("string"), w3995) -> (w3996:string)
            n3082 = Concatenate Strings("1)" ("string"), w4002) -> (w4001:string)
            n3083 = Concatenate Strings("4)" ("string"), w3992) -> (w3993:string)
            n3084 = Concatenate Strings("5)" ("string"), w3990) -> (w3989:string)
            n3085 = Concatenate Strings("6)" ("string"), w3987) -> (w3986:string)
            n3086 = Concatenate Strings("7)" ("string"), w3983) -> (w3984:string)
            n3087 = Concatenate Strings("8)" ("string"), w3980) -> (w3981:string)
            n3088 = local read "HCF 2"() -> (w4019:dbl)
            n3089 = local read "AVP 2"() -> (w4036:dbl)
            n3090 = local read "s.NO"() -> (w3978:string)
            n3091 = call <vilib>:"New Report.vi"("report type"=enum16{"Standard Report", "HTML"}."Standard Report") -> ("report out"=w4057:refnum<class "NI_report.lvclass">, "error out"=w4056:errorcluster)  [unwired: 13 in]
            n3092 = local read "TITTLE"() -> (w4009:string)
            n3093 = Concatenate Strings(w4034, w3977, w3978, w4034, w4012, w4007, w4034, w4011, w4008, w4034, w4013, w4010, w4034) -> (w4027:string)
            "test by" <- w4027
            n3094 = Number To Fractional String(number=w4033, width (-)=i16 6, precision (6)=i16 2) -> (F-format string=w4022:string)  [unwired: 1 in]
            n3095 = Number To Fractional String(number=w4032, width (-)=i16 6, precision (6)=i16 2) -> (F-format string=w4035:string)  [unwired: 1 in]
            n3096 = Number To Fractional String(number=w4048, width (-)=i16 6, precision (6)=i16 2) -> (F-format string=w4053:string)  [unwired: 1 in]
            n3097 = Number To Fractional String(number=w4037, width (-)=i16 6, precision (6)=i16 2) -> (F-format string=w4039:string)  [unwired: 1 in]
            n3098 = Number To Fractional String(number=w4023, width (-)=i16 6, precision (6)=i16 2) -> (F-format string=w4024:string)  [unwired: 1 in]
            n3099 = Number To Fractional String(number=w4036, width (-)=i16 6, precision (6)=i16 2) -> (F-format string=w4038:string)  [unwired: 1 in]
            n3100 = Number To Fractional String(number=w4019, width (-)=i16 6, precision (6)=i16 2) -> (F-format string=w4018:string)  [unwired: 1 in]
            n3101 = Number To Fractional String(number=w4015, precision (6)=i16 2) -> (F-format string=w4014:string)  [unwired: 2 in]
            n3102 = call-dynamic "Set Report Header Text.vi"("report in"=w4057, "center header text"=w4009, "error in (no error)"=w4056) -> ("report out"=w4028:refnum<class "NI_report.lvclass">, "error out"=w4029:errorcluster)  [unwired: 11 in]
            n3103 = Concatenate Strings(w4017, w4001, w4053, w4017, w3998, w4022, w4017, w3996, w4035, w4017, w3993, w4024, w4017, w3989, w4039, w4017, w3986, w4038, w4017, w3984, w4018, w4017, w3981, w4014) -> (w4005:string)
            "export 2" <- w4005
            n3104 = call-poly <vilib>:"Append Report Text.vi"("report in"=w4028, "text"=w4027, "error in (no error)"=w4029) -> ("report out"=w4031:refnum<class "NI_report.lvclass">, "error out"=w4030:errorcluster)  [unwired: 9 in, 2 out]
            n3105 = local read "test by"() -> (w4004:string)
            n3106 = local read "TITTLE"() -> (w4006:string)
            n3107 = call-poly <vilib>:"Append Report Text.vi"("report in"=w4031, "error in (no error)"=w4030) -> ("report out"=w4052:refnum<class "NI_report.lvclass">, "error out"=w4050:errorcluster)  [unwired: 10 in, 2 out]
            n3108 = Concatenate Strings(w4006, w4005, w4004) -> (→"output":string)
            n3109 = call-poly <vilib>:"Append Report Text.vi"("report in"=w4052, "text"=w4005, "error in (no error)"=w4050) -> ("report out"=w4051:refnum<class "NI_report.lvclass">, "error out"=w4049:errorcluster)  [unwired: 9 in, 2 out]
            n3110 = call-dynamic "Print Report.vi"("report in"=w4051, "printer name (default)"=w4059, "error in (no error)"=w4049) -> ("report out"=w4061:refnum<class "NI_report.lvclass">, "error out"=w4062:errorcluster)  [unwired: 11 in]
            n3111 = call-dynamic "Dispose Report.vi"("report in"=w4061, "error in (no error)"=w4062) -> ()  [unwired: 13 in, 1 out]
          }
        }
        n3112 = case shown="True" "Print 2" {
          frame False {
          }
          frame True {
            n3113 = flat-sequence {
              frame #0 {
                n3114 = local read "s.NO"() -> (→"s.NO 2":string)
                n3115 = Wait (ms)(milliseconds to wait=u32 20) -> ()  [unwired: 1 out]
                n3116 = local read "Sample ID  3"() -> (→"Sample ID  6":string)
                n3117 = local read "Sample ID  4"() -> (→"Sample ID  7":string)
                n3118 = local read "Sample ID"() -> (→"Sample ID  2":string)
                n3119 = local read "Tested by"() -> (→"Tested by 2":string)
                n3120 = local read "Test Date"() -> (→"Test Date 2":string)
                n3121 = local read "Humidity after test 3"() -> (→"Humidity after test 4":dbl)
                n3122 = local read "Ref A Test Date :"() -> (→"TITTLE 4":string)
                n3123 = local read "Temperature before test 3"() -> (w3884:dbl)
                n3124 = local read "Temperature before test 3"() -> (→"Temperature after test 5":dbl)
                n3125 = local read "Temperature after test 3"() -> (→"Temperature after test 4":dbl)
                n3126 = local read "Humidity before test 3"() -> (→"Humidity before test 4":dbl)
                n3127 = local write "Temperature before test 3"(w3884) -> ()
                n3128 = local read "image data"() -> (w3875:T16)
                n3129 = String To Path(string="C:\\LAB-IQ\\im\\Temp_resized.jpg") -> (path=w3876:path)
                "path 2" <- w3876
                n3130 = call <vilib>:"Write JPEG File.vi"("image data"=w3875, "path to JPEG file"=w3876) -> ()  [unwired: 8 in, 2 out]
                "Ref A Test Date :" <- "Ref A Test Date :"
                "Ref B Test Date :" <- "Ref B Test Date :"
                "Ref B Scar Value :" <- "Ref B Scar Value :"
                "Ref A Scar Value :" <- "Ref A Scar Value :"
              }
              frame #1 {
                (unwired) HTML_Report_Image_Alignment."MIDDLE" ("alignment (default)")
                w3912 = u16 0 items=["portrait", "landscape"] ("orientation (portrait)")
                (unwired) HTML_Report_Image_Alignment."ABSMIDDLE" ("alignment (default)")
                (unwired) "TESTED BY : "
                (unwired) "TESTED DATE :"
                (unwired) "SAMPLE ID : "
                (unwired) "SAMPLE DESIGN : "
                w3945 = "\r"
                # "add image"
                n3131 = Wait (ms)(milliseconds to wait=u32 20) -> ()  [unwired: 1 out]
                n3132 = local read "Sample ID  2"() -> (w3938:string)
                n3133 = local read "Wear Scar X"() -> (w3910:dbl)
                "Length ( microns ) 2" <- w3910
                n3134 = local read "Wear Scar Y"() -> (w3909:dbl)
                "Wear Scar Y ( microns ) :" <- w3909
                n3135 = local read "Test Date 2"() -> (w3939:string)
                n3136 = local read "Tested by 2"() -> (w3940:string)
                n3137 = local read "String 46"() -> (w3936:string)
                n3138 = local read "String 48"() -> (w3942:string)
                n3139 = local read "String 47"() -> (w3941:string)
                n3140 = local read "String 49"() -> (w3943:string)
                n3141 = local read "String 10"() -> (w3896:string)
                n3142 = local read "s.NO 2"() -> (w3937:string)
                n3143 = Add(x=w3910, y=w3909) -> (x+y=w3908:dbl)
                n3144 = call <vilib>:"New Report.vi"("report type"=enum16{"Standard Report", "HTML"}."HTML") -> ("report out"=w3916:refnum<class "NI_report.lvclass">, "error out"=w3914:errorcluster)  [unwired: 13 in]
                n3145 = Concatenate Strings(w3945, w3936, w3937, w3945, w3942, w3938, w3945, w3941, w3939, w3945, w3943, w3940, w3945) -> (→"test by 2":string)
                n3146 = Concatenate Strings("C:\\LAB-IQ\\Data\\" ("string"), w3896, ".jpg" ("string")) -> ()  [unwired: 1 out]
                n3147 = Divide(x=w3908, y=2.0) -> (x/y=→"Mean Wear ( microns) :":dbl)
                n3148 = call-dynamic "Set Report Orientation.vi"("report in"=w3916, "orientation (portrait)"=w3912, "error in (no error)"=w3914) -> ("report out"=w3915:refnum<class "NI_report.lvclass">, "error out"=w3913:errorcluster)  [unwired: 11 in]
                n3149 = for {
                  N: 5 -> [_]
                  tunnel: w3915 -> [w3966]
                  tunnel: [w3965] -> w3894
                  tunnel: w3913 -> [w3964]
                  tunnel: [w3963] -> w3893
                  n3150 = call-dynamic "Set Report Tab Width.vi"("report in"=w3966, "error in (no error)"=w3964) -> ("report out"=w3965:refnum<class "NI_report.lvclass">, "error out"=w3963:errorcluster)  [unwired: 12 in]
                }
                n3151 = local read "TITTLE"() -> (w3911:string)
                n3152 = call-dynamic "Set Report Header Text.vi"("report in"=w3894, "center header text"=w3911, "error in (no error)"=w3893) -> ("report out"=w3932:refnum<class "NI_report.lvclass">, "error out"=w3931:errorcluster)  [unwired: 11 in]